vi "ScanDelay_FTIR_BBnorm_Aligning_NewportFlipper.vi"() -> ()   [LabVIEW 2022 SP3] (continued)
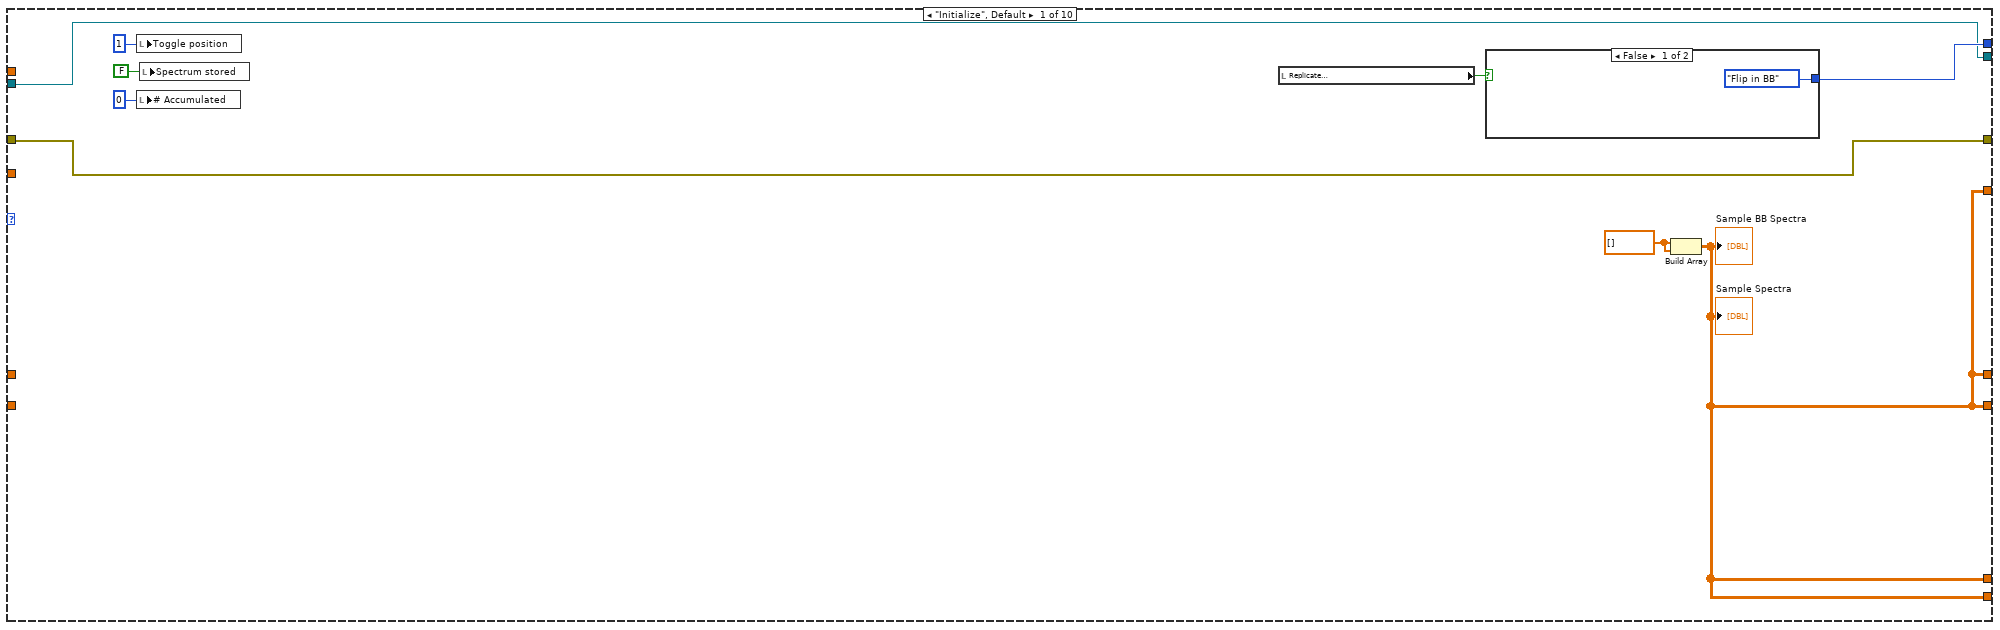
[diagram p3: hidden frame]
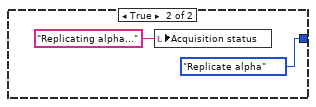
[diagram p4: hidden frame]
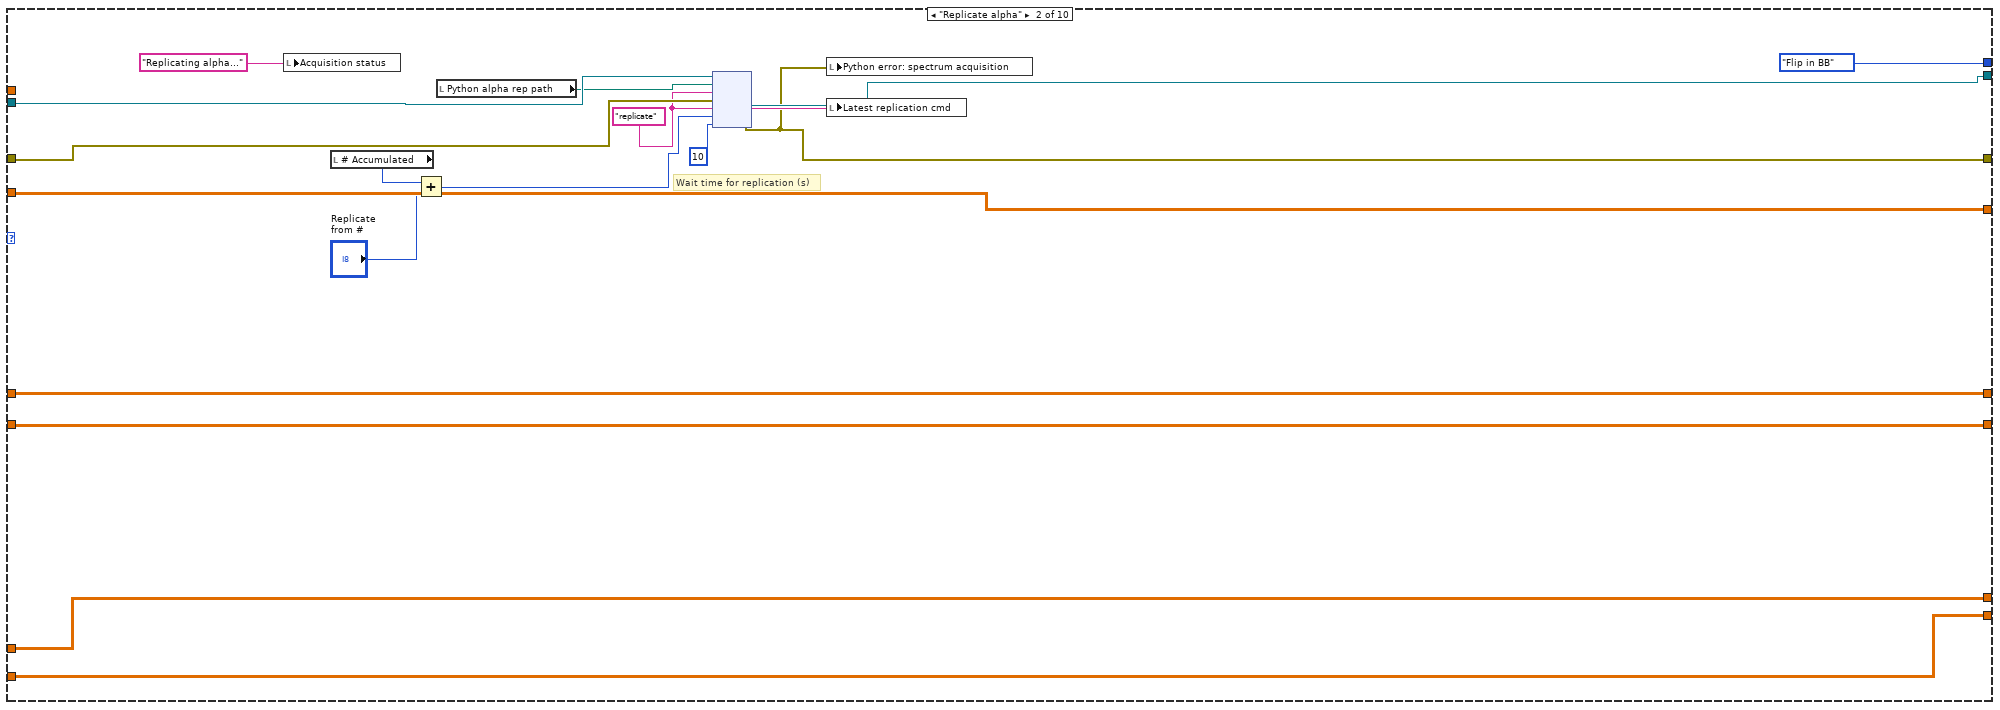
[diagram p5: hidden frame]
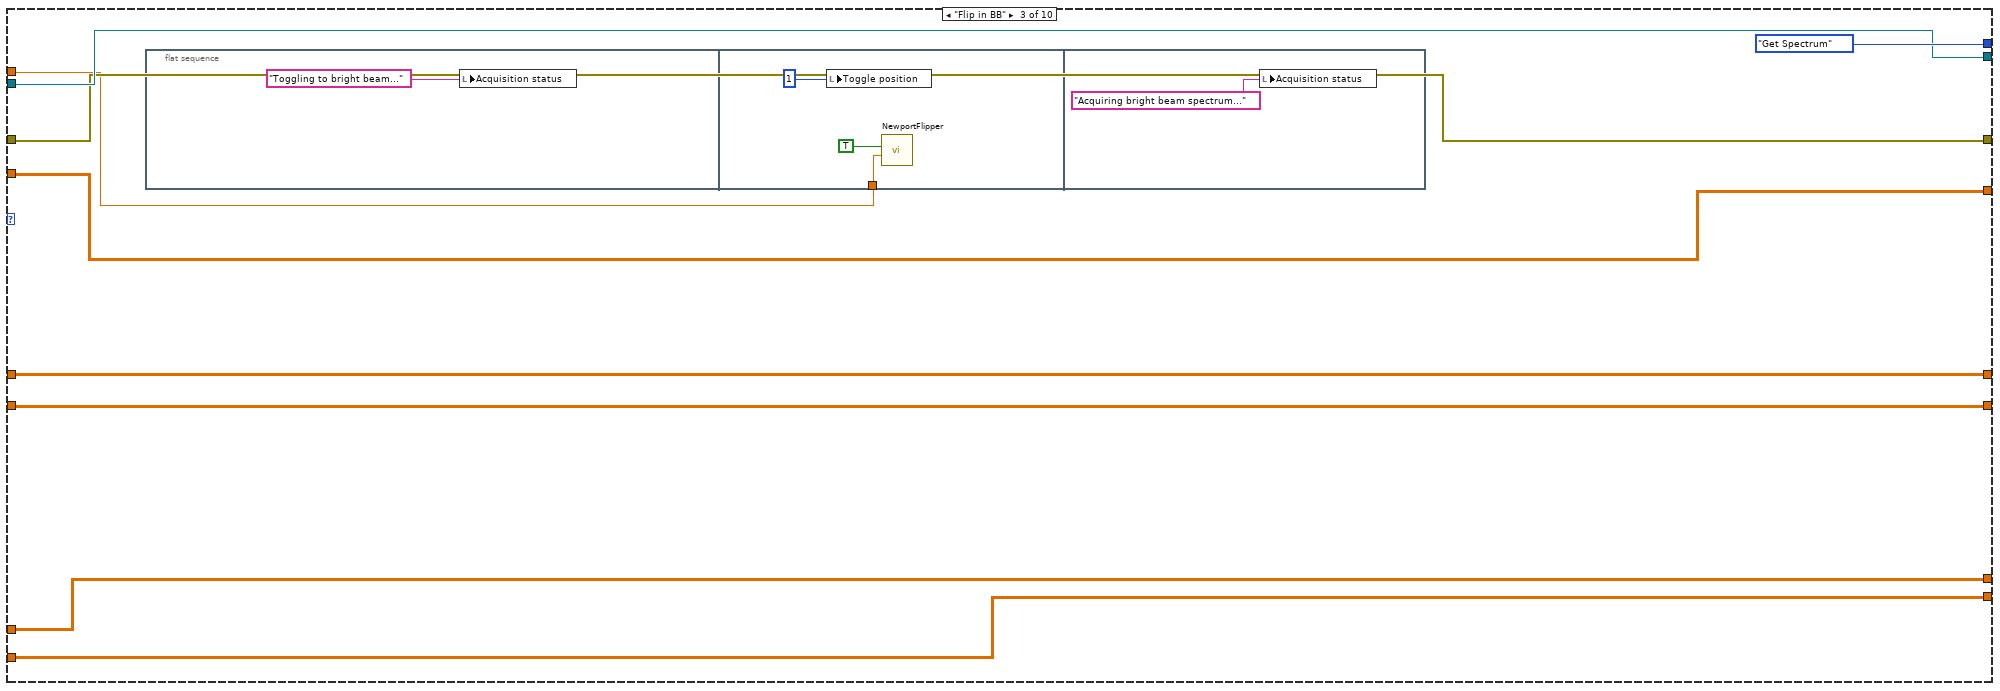
[diagram p6: hidden frame]
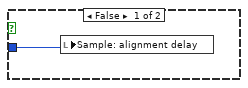
[diagram p8: hidden frame]
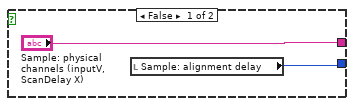
[diagram p9: hidden frame]
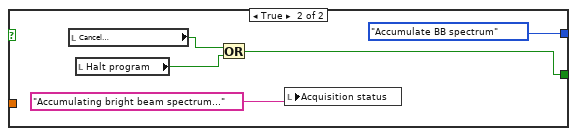
[diagram p11: hidden frame]
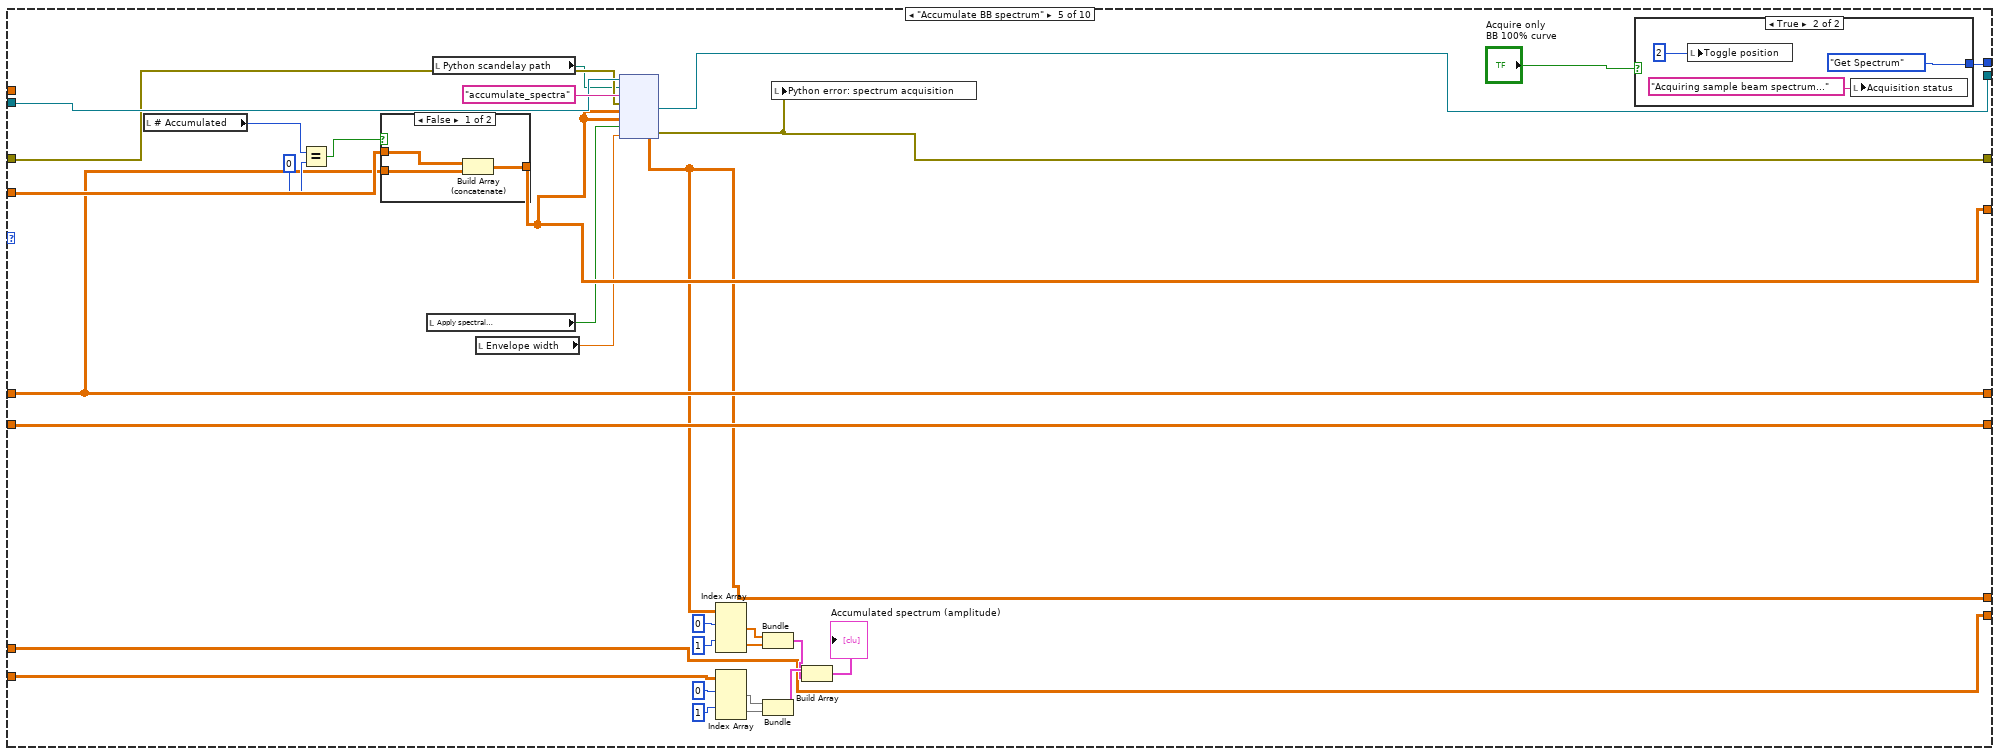
[diagram p12: hidden frame]
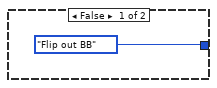
[diagram p13: hidden frame]
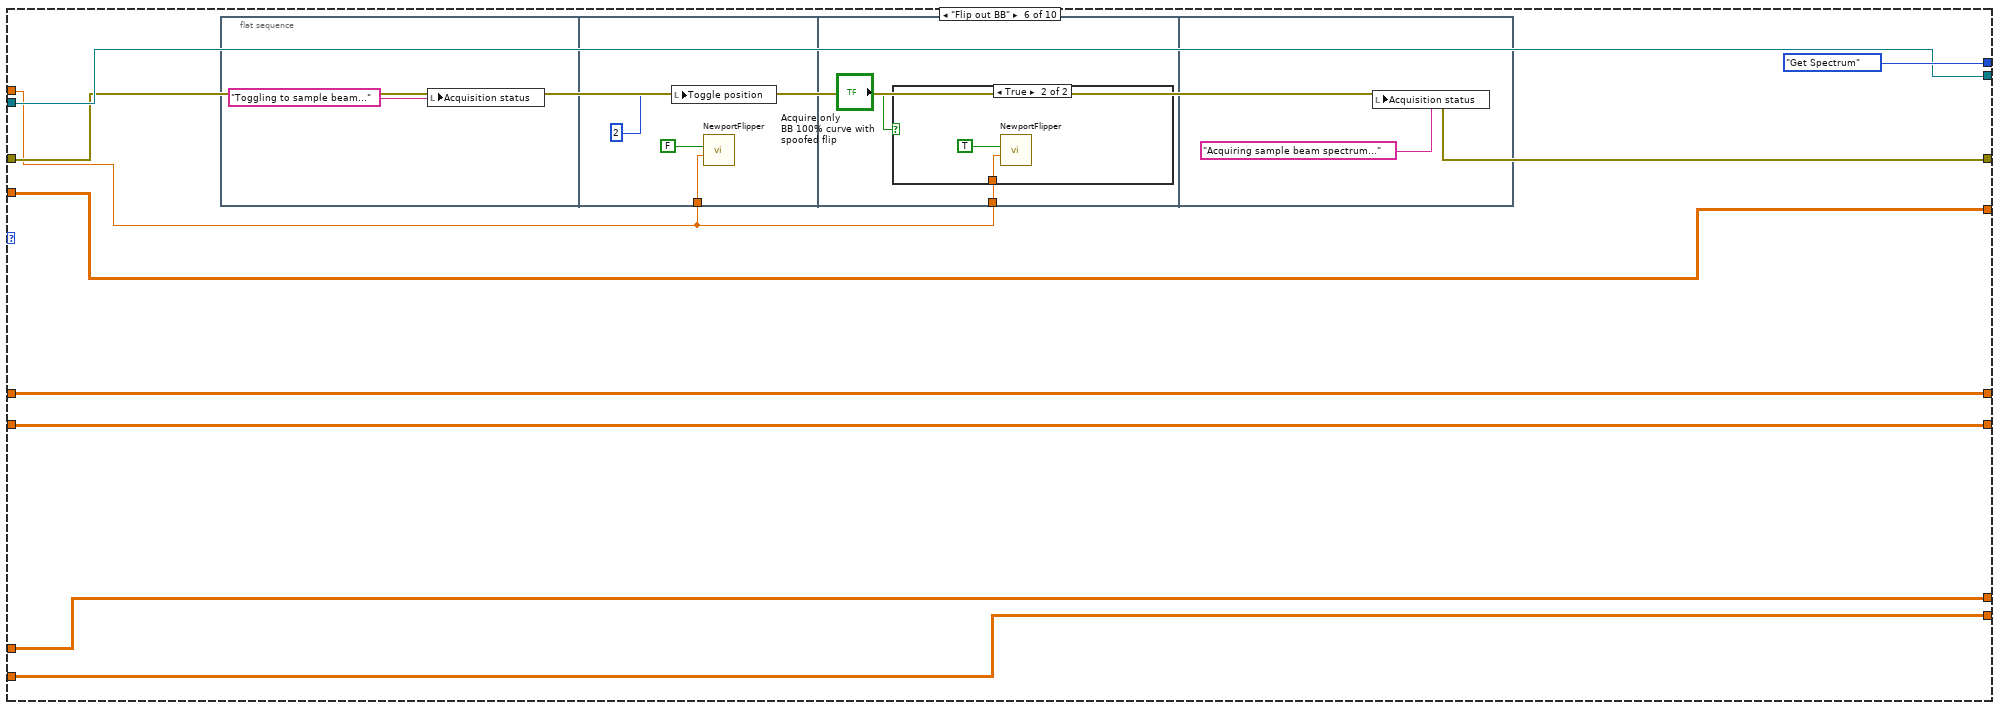
[diagram p15: hidden frame]
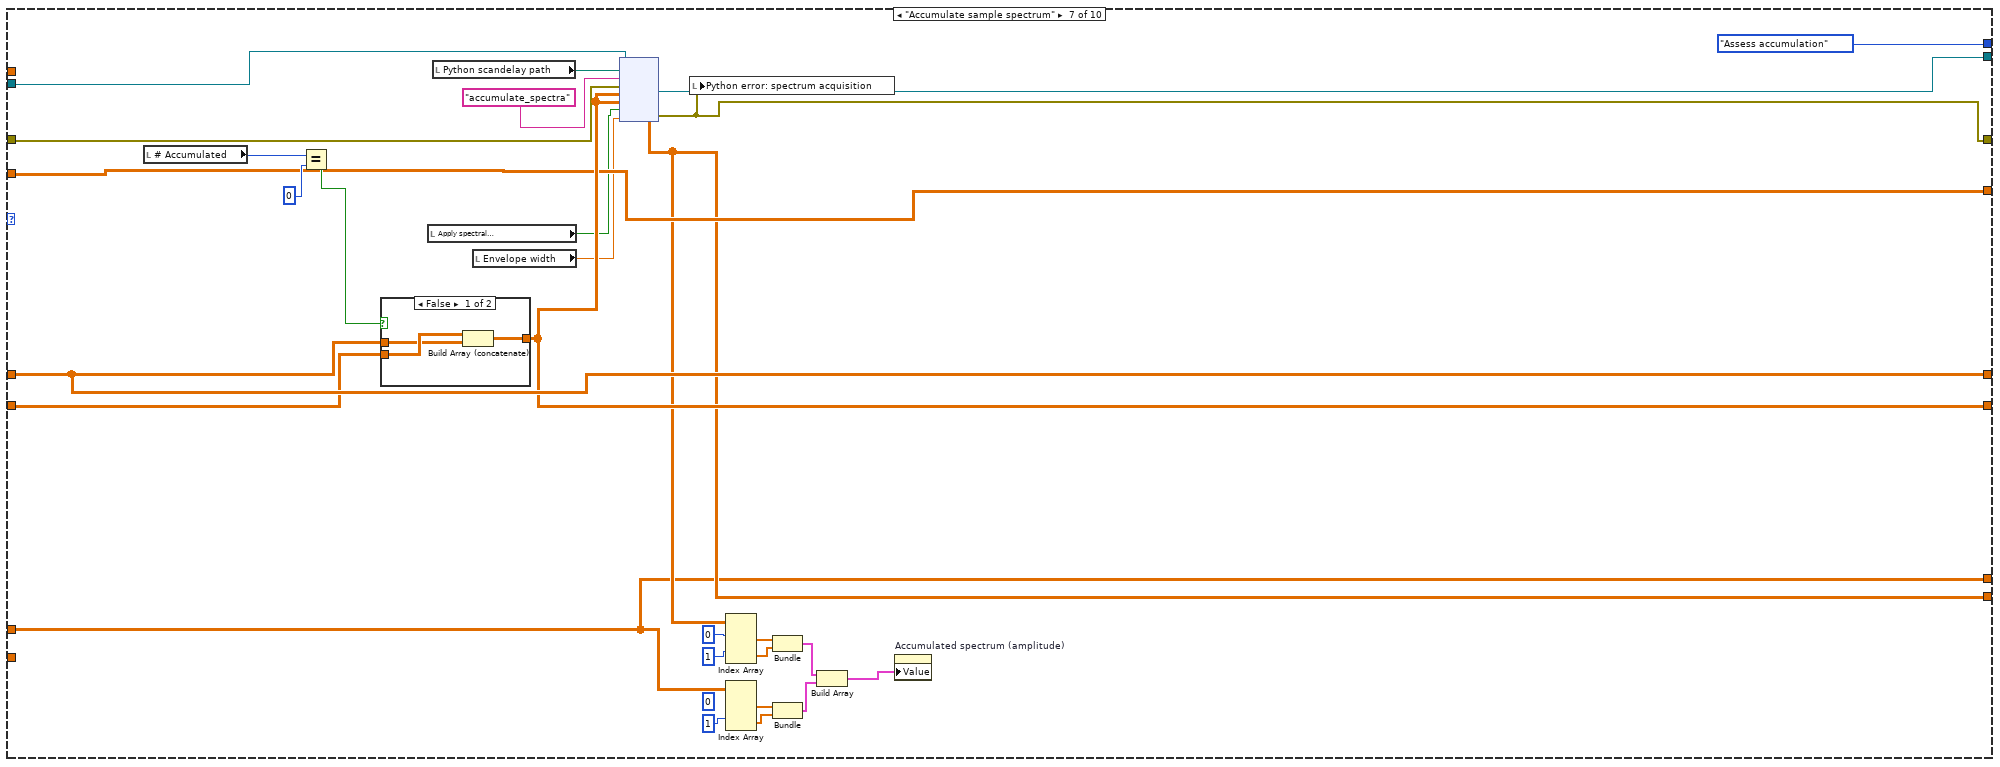
[diagram p17: hidden frame]
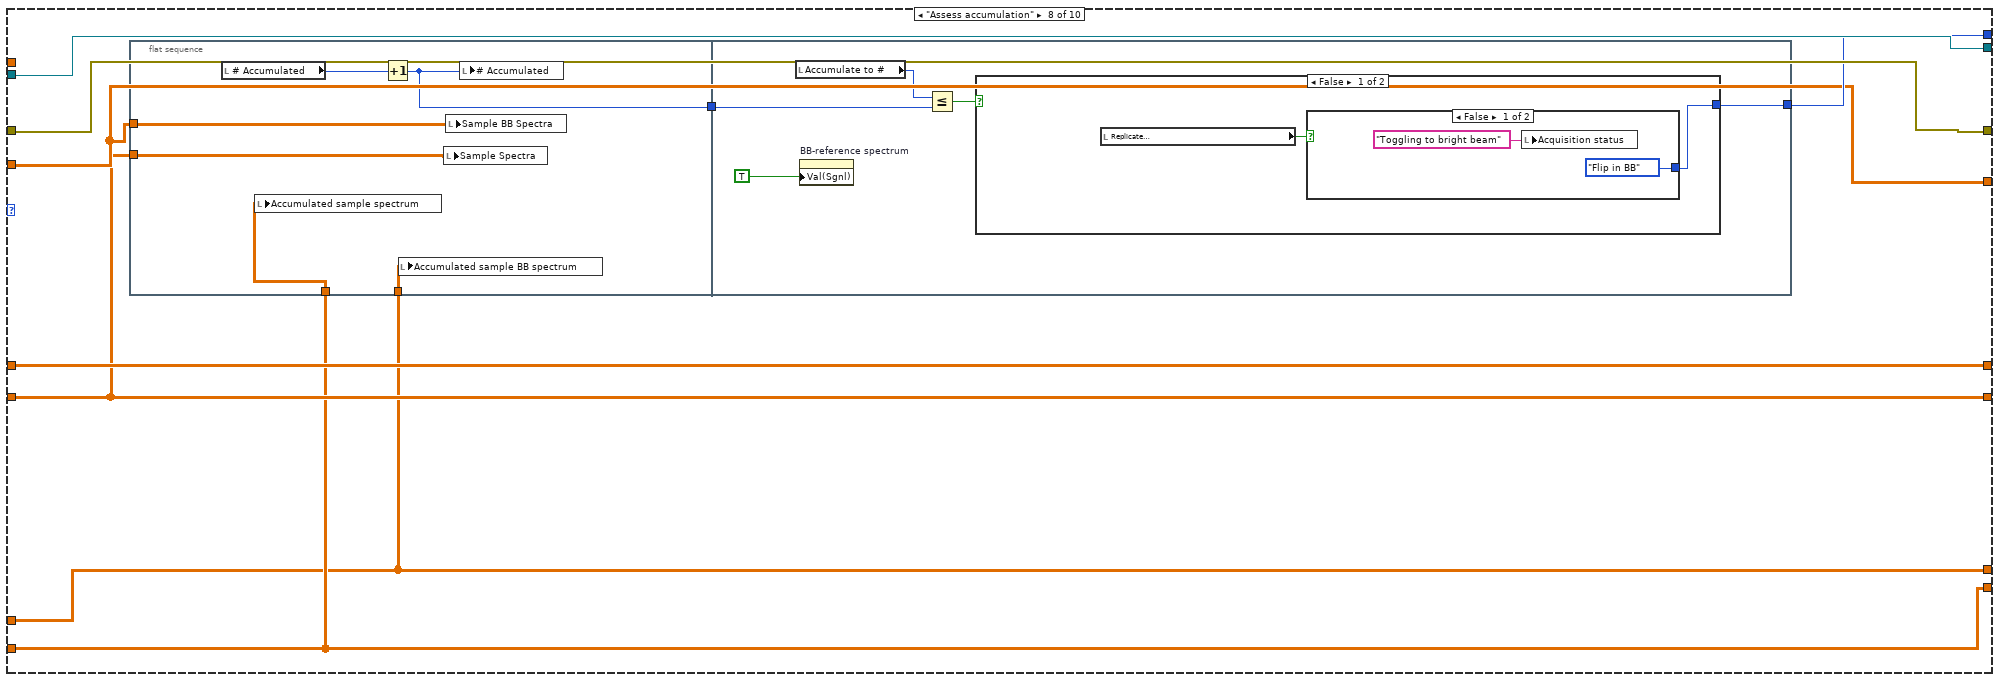
[diagram p19: hidden frame]
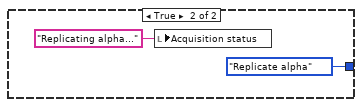
[diagram p20: hidden frame]
            tunnel: w324 -> [_ w363 w369 w404 w434 w471 w496 w517 w544 w555]
            tunnel: [w342 Control_GetSpectrum_BBnorm."Flip in BB" Control_GetSpectrum_BBnorm."Get Spectrum" w387 w441 Control_GetSpectrum_BBnorm."Get Spectrum" Control_GetSpectrum_BBnorm."Assess accumulation" w520 Control_GetSpectrum_BBnorm."Done" Control_GetSpectrum_BBnorm."Done"] -> w323
            tunnel: w322 -> [w339 w360 w372 w398 w451 w470 w506 w522 w546 w559]
            tunnel: w321 -> [w338 w359 w371 w405 w450 w469 w505 w523 w545 w558]
            tunnel: [w338 w353 w371 w405 w440 w469 w494 w523 w545 w558] -> w320
            tunnel: [w339 w354 w372 w398 w449 w470 w504 w522 w546 w559] -> w319
            tunnel: [w335 w352 w368 w390 w442 w468 w498 w519 w550 w556] -> w318
            tunnel: w316 -> [_ w352 w368 _ w442 w468 w498 w519 w550 w556]
            tunnel: "Toggle pause (ms)" -> [_ _ w365 _ _ w465 _ _ _ _]
            tunnel: [w335 w351 w367 w400 w430 w467 w485 w515 w548 w553] -> w314
            tunnel: [w335 w350 w366 w399 w428 w466 w486 w516 w547 w552] -> w313
            tunnel: w312 -> [_ w351 w367 w400 w428 w467 w485 w515 w548 w553]
            tunnel: w311 -> [_ w350 w366 w399 w429 w466 _ w516 w547 w552]
            frame "Initialize", Default {
              w343 = dbl[] []
              n175 = local write "Toggle position"(1) -> ()
              n176 = local write "# Accumulated"(0) -> ()
              n177 = local write "Spectrum stored"(FALSE) -> ()
              n178 = local read "Replicate\nalpha on\naccumulation"() -> (w340:bool)
              n179 = case shown="False" w340 {
                tunnel: [Control_GetSpectrum_BBnorm."Flip in BB" Control_GetSpectrum_BBnorm."Replicate alpha"] -> w342
                frame False {
                }
                frame True {
                  n180 = local write "Acquisition status"("Replicating alpha...") -> ()
                }
              }
              n181 = Build Array(w343, w343) -> (w335:dbl[][])
              "Sample Spectra" <- w335
              "Sample BB Spectra" <- w335
            }
            frame "Replicate alpha" {
              w357 = "replicate"
              # "Wait time for replication (s)"
              n182 = local write "Acquisition status"("Replicating alpha...") -> ()
              n183 = local read "# Accumulated"() -> (w349:i32)
              n184 = Add(x=w349, y="Replicate\nfrom #") -> (x+y=w347:i32)
              n185 = local read "Python alpha rep path"() -> (w358:path)
              n186 = node(w360, w358, w357, w359, w357, w347, 10) -> (w354:refnum<k35>, w353:errorcluster, w355:string)  [unwired: 2 in, 2 out]
              n187 = local write "Python error: spectrum acquisition"(w353) -> ()
              n188 = local write "Latest replication cmd"(w355) -> ()
            }
            frame "Flip in BB" {
              n189 = flat-sequence {
                tunnel: w365 -> [w375]
                frame #0 {
                  n190 = local write "Acquisition status"("Toggling to bright beam...") -> ()
                }
                frame #1 {
                  n191 = local write "Toggle position"(1) -> ()
                  n192 = call "NewportFlipper.vi"("Settle time (ms)"=w375, "Up/Down"=TRUE) -> ()  [unwired: 10 in]
                }
                frame #2 {
                  n193 = local write "Acquisition status"("Acquiring bright beam spectrum...") -> ()
                }
              }
            }
            frame "Get Spectrum" {
              n194 = control-ref of="% averaged"() -> (w396:refnum<vi>)
              n195 = control-ref of="Acquisition cycle"() -> (w395:refnum<vi>)
              n196 = control-ref of="Cancel\nacquisition"() -> (w389:refnum<vi>)
              n197 = local read "Toggle position"() -> (w402:i32)
              n198 = control-ref of="Binned interferogram"() -> (w397:refnum<vi>)
              n199 = Equal?(x=w402, y=1) -> (x = y?=w382:bool)
              n200 = case shown="True" w382 {
                tunnel: ["Sample: physical channels (inputV, ScanDelay X)" "Bright beam: physical channels (inputV, ScanDelay X)"] -> w384
                tunnel: [w410 w412] -> w383
                frame False {
                  n201 = local read "Sample: alignment delay"() -> (w410:i32)
                }
                frame True {
                  n202 = local read "Bright beam: alignment delay"() -> (w412:i32)
                }
              }
              n203 = call "ScanDelay_FTIR_GetSpectrum_Aligning.vi"("Cancel? External"=w389, "% averaged (external)"=w396, "Binned interferogram (external)"=w397, "Python refnum in"=w398, "Optimize\ninterferogram\ndelay"="Optimize\ninterferogram\nalignment", "Acquisition cycle (external)"=w395, "Displacement\n calibration  factor"="Delay calibratior\nfactor (ps/V)", "Channels to read (input V, ScanDelay)"=w384, "Acquisitions per interferogram"="Cycles per\ninterferogram", "Time per\nacquisition (s)"="Time per\nacquisition (s)", "Sampling rate"="Sampling rate", "Delay estimation (pts)"=w383) -> ("Output spectrum"=w390:dbl[][], "Best delay"=w385:i32)  [unwired: 2 in]
              n204 = And(x="Optimize\ninterferogram\nalignment", y="Update alignment") -> (x .and. y?=w379:bool)
              n205 = case shown="True" w379 {
                tunnel: w385 -> [_ w407]
                tunnel: w382 -> [_ w406]
                frame False {
                }
                frame True {
                  # "Update our optimal delay only if we are actively optimizing"
                  n206 = case shown="True" w406 {
                    tunnel: w407 -> [w408 w409]
                    frame False {
                      n207 = local write "Sample: alignment delay"(w408) -> ()
                    }
                    frame True {
                      n208 = local write "Bright beam: alignment delay"(w409) -> ()
                    }
                  }
                }
              }
              n209 = case shown="False" w382 {
                tunnel: [Control_GetSpectrum_BBnorm."Accumulate sample spectrum" Control_GetSpectrum_BBnorm."Accumulate BB spectrum"] -> w388
                tunnel: w390 -> [_ _]
                tunnel: [w416 w421] -> w386
                frame False {
                  n210 = local read "Cancel\nacquisition"() -> (w417:bool)
                  n211 = local read "Halt program"() -> (w418:bool)
                  n212 = Or(x=w417, y=w418) -> (x .or. y?=w416:bool)
                  n213 = local write "Acquisition status"("Accumulating sample spectrum...") -> ()
                }
                frame True {
                  n214 = local read "Cancel\nacquisition"() -> (w423:bool)
                  n215 = local read "Halt program"() -> (w422:bool)
                  n216 = Or(x=w423, y=w422) -> (x .or. y?=w421:bool)
                  n217 = local write "Acquisition status"("Accumulating bright beam spectrum...") -> ()
                }
              }
              n218 = case shown="True" w386 {
                tunnel: w388 -> [w414 _]
                tunnel: [w414 Control_GetSpectrum_BBnorm."Done"] -> w387
                frame False {
                }
                frame True {
                }
              }
            }
            frame "Accumulate BB spectrum" {
              n219 = local read "# Accumulated"() -> (w455:i32)
              n220 = Equal?(x=w455, y=0) -> (x = y?=w453:bool)
              n221 = case shown="False" w453 {
                tunnel: w442 -> [w462 w464]
                tunnel: w456 -> [w463 _]
                tunnel: [w461 w464] -> w447
                frame False {
                  n222 = Build Array (concatenate)(w463, w462) -> (w461:dbl[][])
                }
                frame True {
                }
              }
              n223 = local read "Apply spectral\nenvelope"() -> (w427:bool)
              n224 = local read "Python scandelay path"() -> (w448:path)
              n225 = local read "Envelope width"() -> (w426:dbl)
              n226 = node(w451, w448, "accumulate_spectra", w450, w447, w447, w427, w426) -> (w449:refnum<k35>, w440:errorcluster, w430:dbl[][])  [unwired: 3 in, 2 out]
              n227 = Index Array(array=w430, index (row) #1=0, index (row) #2=1) -> (element #1=w444:dbl[], element #2=w443:dbl[])  [unwired: 2 in]
              n228 = Index Array(array=w429, index (row) #1=0, index (row) #2=1) -> (element #1=w436:dbl[], element #2=w435:dbl[])  [unwired: 2 in]
              n229 = Bundle("Output spectrum"=w444, "Output spectrum"=w443) -> (w432:T1)  [unwired: 1 in]
              n230 = Bundle("Output spectrum"=w436, "Output spectrum"=w435) -> (w433:T1)  [unwired: 1 in]
              n231 = local write "Python error: spectrum acquisition"(w440) -> ()
              n232 = Build Array(w433, w432) -> (→"Accumulated spectrum (amplitude)":T3)
              n233 = case shown="True" "Acquire only\nBB 100% curve" {
                tunnel: [Control_GetSpectrum_BBnorm."Flip out BB" Control_GetSpectrum_BBnorm."Get Spectrum"] -> w441
                frame False {
                }
                frame True {
                  n234 = local write "Toggle position"(2) -> ()
                  n235 = local write "Acquisition status"("Acquiring sample beam spectrum...") -> ()
                }
              }
            }
            frame "Flip out BB" {
              n236 = flat-sequence {
                tunnel: w465 -> [w475]
                tunnel: w465 -> [w478]
                frame #0 {
                  n237 = local write "Acquisition status"("Toggling to sample beam...") -> ()
                }
                frame #1 {
                  n238 = local write "Toggle position"(2) -> ()
                  n239 = call "NewportFlipper.vi"("Settle time (ms)"=w475, "Up/Down"=FALSE) -> ()  [unwired: 10 in]
                }
                frame #2 {
                  n240 = case shown="True" "Acquire only\nBB 100% curve with\nspoofed flip" {
                    tunnel: w478 -> [_ w480]
                    frame False {
                    }
                    frame True {
                      n241 = call "NewportFlipper.vi"("Settle time (ms)"=w480, "Up/Down"=TRUE) -> ()  [unwired: 10 in]
                    }
                  }
                }
                frame #3 {
                  n242 = local write "Acquisition status"("Acquiring sample beam spectrum...") -> ()
                }
              }
            }
            frame "Accumulate sample spectrum" {
              (unwired) 0
              n243 = local read "# Accumulated"() -> (w510:i32)
              n244 = Equal?(x=w510, y=0) -> (x = y?=w508:bool)
              n245 = case shown="False" w508 {
                tunnel: w498 -> [w512 w514]
                tunnel: w496 -> [w513 _]
                tunnel: [w511 w514] -> w495
                frame False {
                  n246 = Build Array (concatenate)(w513, w512) -> (w511:dbl[][])
                }
                frame True {
                }
              }
              n247 = local read "Apply spectral\nenvelope"() -> (w484:bool)
              n248 = local read "Python scandelay path"() -> (w503:path)
              n249 = local read "Envelope width"() -> (w483:dbl)
              n250 = node(w506, w503, "accumulate_spectra", w505, w495, w495, w484, w483) -> (w504:refnum<k35>, w494:errorcluster, w486:dbl[][])  [unwired: 3 in, 2 out]
              n251 = local write "Python error: spectrum acquisition"(w494) -> ()
              n252 = Index Array(array=w486, index (row) #1=0, index (row) #2=1) -> (element #1=w500:dbl[], element #2=w499:dbl[])  [unwired: 2 in]
              n253 = Index Array(array=w485, index (row) #2=1) -> (element #1=w491:dbl[], element #2=w490:dbl[])  [unwired: 3 in]
              n254 = Bundle("Output spectrum"=w500, "Output spectrum"=w499) -> (w493:T1)  [unwired: 1 in]
              n255 = Bundle("Output spectrum"=w491, "Output spectrum"=w490) -> (w489:T1)  [unwired: 1 in]
              n256 = Build Array(w493, w489) -> (w487:T3)
              n257 = property on="Accumulated spectrum (amplitude)" class="XYGraph (strict)"("Value"=w487) -> ()  [unwired: 2 in, 2 out]
            }
            frame "Assess accumulation" {
              n258 = flat-sequence {
                tunnel: [w528] -> w521
                tunnel: w518 -> [w527]
                tunnel: w517 -> [w526]
                tunnel: w516 -> [w524]
                tunnel: w515 -> [w525]
                tunnel: w521 -> [w530]
                tunnel: [w534] -> w520
                frame #0 {
                  n259 = local read "# Accumulated"() -> (w529:i32)
                  n260 = local write "Accumulated sample spectrum"(w524) -> ()
                  n261 = Increment(x=w529) -> (x+1=w528:i32)
                  n262 = local write "Accumulated sample BB spectrum"(w525) -> ()
                  n263 = local write "Sample Spectra"(w526) -> ()
                  n264 = local write "Sample BB Spectra"(w527) -> ()
                  n265 = local write "# Accumulated"(w528) -> ()
                }
                frame #1 {
                  n266 = local read "Accumulate to #"() -> (w531:i32)
                  n267 = property on="BB-reference spectrum" class="Bool (strict)"("Val(Sgnl)"=TRUE) -> ()  [unwired: 2 in, 2 out]
                  n268 = Less Or Equal?(x=w531, y=w530) -> (x <= y?=w532:bool)
                  n269 = case shown="False" w532 {
                    tunnel: [w535 Control_GetSpectrum_BBnorm."Finalize"] -> w534
                    frame False {
                      n270 = local read "Replicate\nalpha on\naccumulation"() -> (w536:bool)
                      n271 = case shown="False" w536 {
                        tunnel: [Control_GetSpectrum_BBnorm."Flip in BB" Control_GetSpectrum_BBnorm."Replicate alpha"] -> w535
                        frame False {
                          n272 = local write "Acquisition status"("Toggling to bright beam") -> ()
                        }
                        frame True {
                          n273 = local write "Acquisition status"("Replicating alpha...") -> ()
                        }
                      }
                    }
                    frame True {
                    }
                  }
                }
              }
            }
            frame "Finalize" {
              n274 = local write "Spectrum stored"(TRUE) -> ()
            }
            frame "Done" {
              w551 = FALSE
              n275 = local write "Acquire spectrum"(w551) -> ()
              n276 = local write "Cancel\nacquisition"(w551) -> ()
            }
          }
          n277 = Wait (ms)(milliseconds to wait=5) -> ()  [unwired: 1 out]
        }
      }
      event Timeout {
        n278 = event-data() -> ()  [unwired: 1 in, 3 out]
        n279 = Wait (ms)(milliseconds to wait=w562) -> ()  [unwired: 1 out]
      }
    }
    n280 = Wait (ms)(milliseconds to wait=5) -> ()  [unwired: 1 out]
    n281 = local read "Halt program"() -> (w301:bool)
    "Acquisition status" <- "Ready to acquire spectrum"
  }
  n282 = Close Python Session(session in=w13, error in=w12) -> (11:w9:errorcluster)
  n283 = local write "Python error: activity loop"(w9) -> ()
  n284 = Close Python Session(session in=w3, error in=w2) -> ()  [unwired: 1 out]
